vi "TLB Native Dynamic Events ver 0.26.vi"() -> ()   [LabVIEW 2018] (continued)
                      tunnel: string[] ["DISPOSE BUFFERS", "READ STEPPER VALUES", ""] -> [w1790] mode=indexing
                      n604 = Enqueue Element(queue=w1792, element=w1790) -> (queue out=w1791:refnum<queue>)  [unwired: 2 in, 2 out]
                    }
                  }
                }
                n605 = Or(x=w1770, y=w1775) -> (x .or. y?=w1777:bool)
                n606 = Select(t=State_Type_Definitions,_for_0.26g_versions_and_later_2."True Stop" ("Enum"), s=w1775, f=State_Type_Definitions,_for_0.26g_versions_and_later_2."Task 8I: ARM GRAB HEIGHT" ("Enum")) -> (s? t:f=w1772:T16)
                n607 = Select(t=w1772, s=w1777, f=State_Type_Definitions,_for_0.26g_versions_and_later_2."Task 8H: ARM ADJUST" ("Enum")) -> (s? t:f=w1776:T16)
              }
              frame "Exit" {
                n608 = for {
                  shift-right: [w1799] -> w1796
                  shift-left: w1793 -> [w1800]
                  tunnel: string[] ["STOP", "RESET ENCODERS", "RESET YAW", "ARDUINO MODE 0"] -> [w1798] mode=indexing
                  n609 = Enqueue Element(queue=w1800, element=w1798) -> (queue out=w1799:refnum<queue>)  [unwired: 2 in, 2 out]
                }
              }
            }
            n610 = Bundle By Name(cluster=w1759, "yStepper desired"=w1755) -> (w1758:T18)
          }
          frame 35 {
            # ">>> Motor control cluster >>>"
            # ">>> yStepper command>>>"
            # ">> Manual override >>"
            n611 = Dequeue Element(queue=w1811, timeout in ms (-1)=w1810, error in (no error)=w1812) -> (element=w1809:T8)  [unwired: 3 out]
            n612 = Equal?(x=w1808, y=u8 1) -> (x = y?=w1806:bool)
            n613 = case shown="\"Start Task 1\", Default" w1809 {
              tunnel: [w1822 State_Type_Definitions,_for_0.26g_versions_and_later_2."True Stop" ("Enum")] -> w1813
              tunnel: [w1825 w1842] -> w1814
              tunnel: [State_Type_Definitions,_for_0.26g_versions_and_later_2."Idle" ("Enum") State_Type_Definitions,_for_0.26g_versions_and_later_2."Shutdown" ("Enum")] -> w1815
              tunnel: w1806 -> [w1821 _]
              tunnel: w1805 -> [w1820 _]
              tunnel: w1804 -> [w1816 w1839]
              frame "Start Task 1", Default {
                # "Stays in Task 5F until stepper reaches desired \nheight"
                # "T: Go back to idle, F: Continue with task\""
                # ">> Manual override >>"
                n614 = case shown="True" w1821 {
                  tunnel: [w1829 w1835] -> w1825
                  tunnel: w1816 -> [w1827 w1833]
                  frame False {
                    n615 = for {
                      tunnel: string[] ["Z STEPPER GRAB HEIGHT", "READ STEPPER VALUES"] ("element") -> [w1830] mode=indexing
                      shift-right: [w1832] -> w1829
                      shift-left: w1827 -> [w1831]
                      n616 = Enqueue Element(queue=w1831, element=w1830) -> (queue out=w1832:refnum<queue>)  [unwired: 2 in, 2 out]
                    }
                  }
                  frame True {
                    n617 = for {
                      shift-right: [w1837] -> w1835
                      shift-left: w1833 -> [w1838]
                      tunnel: string[] ["SET TIMER 2", "CLOSE CLAW", ""] -> [w1836] mode=indexing
                      n618 = Enqueue Element(queue=w1838, element=w1836) -> (queue out=w1837:refnum<queue>)  [unwired: 2 in, 2 out]
                    }
                  }
                }
                n619 = Or(x=w1821, y=w1820) -> (x .or. y?=w1823:bool)
                n620 = Select(t=State_Type_Definitions,_for_0.26g_versions_and_later_2."True Stop" ("Enum"), s=w1820, f=State_Type_Definitions,_for_0.26g_versions_and_later_2."Task 8J: CLOSE CLAW" ("Enum")) -> (s? t:f=w1817:T16)
                n621 = Select(t=w1817, s=w1823, f=State_Type_Definitions,_for_0.26g_versions_and_later_2."Task 8I: ARM GRAB HEIGHT" ("Enum")) -> (s? t:f=w1822:T16)
              }
              frame "Exit" {
                n622 = for {
                  shift-right: [w1845] -> w1842
                  shift-left: w1839 -> [w1846]
                  tunnel: string[] ["STOP", "RESET ENCODERS", "RESET YAW", "ARDUINO MODE 0"] -> [w1844] mode=indexing
                  n623 = Enqueue Element(queue=w1846, element=w1844) -> (queue out=w1845:refnum<queue>)  [unwired: 2 in, 2 out]
                }
              }
            }
          }
          frame 36 {
            # ">>> yStepper command>>>"
            # ">> Manual override >>"
            n624 = Dequeue Element(queue=w1857, timeout in ms (-1)=w1856, error in (no error)=w1855) -> (element=w1854:T8)  [unwired: 3 out]
            n625 = case shown="\"Start Task 1\", Default" w1854 {
              tunnel: [w1866 State_Type_Definitions,_for_0.26g_versions_and_later_2."True Stop" ("Enum")] -> w1859
              tunnel: [w1869 w1886] -> w1852
              tunnel: [State_Type_Definitions,_for_0.26g_versions_and_later_2."Idle" ("Enum") State_Type_Definitions,_for_0.26g_versions_and_later_2."Shutdown" ("Enum")] -> w1851
              tunnel: w1853 -> [w1860 _]
              tunnel: w1858 -> [w1865 w1883]
              tunnel: w1849 -> [w1864 _]
              frame "Start Task 1", Default {
                # ">> Is time up? >>"
                # "Determines if object is in range to pick up"
                # ">> Manual override >>"
                n626 = case shown="True" w1864 {
                  tunnel: [w1873 w1879] -> w1869
                  tunnel: w1865 -> [w1871 w1877]
                  frame False {
                    n627 = for {
                      tunnel: string[] ["CLOSE CLAW", "START TIMER"] ("element") -> [w1874] mode=indexing
                      shift-right: [w1876] -> w1873
                      shift-left: w1871 -> [w1875]
                      n628 = Enqueue Element(queue=w1875, element=w1874) -> (queue out=w1876:refnum<queue>)  [unwired: 2 in, 2 out]
                    }
                  }
                  frame True {
                    n629 = for {
                      shift-right: [w1881] -> w1879
                      shift-left: w1877 -> [w1882]
                      tunnel: string[] ["READ STEPPER VALUES", "", ""] -> [w1880] mode=indexing
                      n630 = Enqueue Element(queue=w1882, element=w1880) -> (queue out=w1881:refnum<queue>)  [unwired: 2 in, 2 out]
                    }
                  }
                }
                n631 = Or(x=w1864, y=w1860) -> (x .or. y?=w1867:bool)
                n632 = Select(t=State_Type_Definitions,_for_0.26g_versions_and_later_2."True Stop" ("Enum"), s=w1860, f=State_Type_Definitions,_for_0.26g_versions_and_later_2."Task 8K: RAISE MY SWORD" ("Enum")) -> (s? t:f=w1862:T16)
                n633 = Select(t=w1862, s=w1867, f=State_Type_Definitions,_for_0.26g_versions_and_later_2."Task 8J: CLOSE CLAW" ("Enum")) -> (s? t:f=w1866:T16)
              }
              frame "Exit" {
                n634 = for {
                  shift-right: [w1889] -> w1886
                  shift-left: w1883 -> [w1890]
                  tunnel: string[] ["STOP", "RESET ENCODERS", "RESET YAW", "ARDUINO MODE 0"] -> [w1888] mode=indexing
                  n635 = Enqueue Element(queue=w1890, element=w1888) -> (queue out=w1889:refnum<queue>)  [unwired: 2 in, 2 out]
                }
              }
            }
          }
          frame 37 {
            # ">>> yStepper command>>>"
            # ">> Manual override >>"
            n636 = Dequeue Element(queue=w1901, timeout in ms (-1)=w1900, error in (no error)=w1902) -> (element=w1899:T8)  [unwired: 3 out]
            n637 = Equal?(x=w1898, y=u8 60) -> (x = y?=w1896:bool)
            n638 = case shown="\"Start Task 1\", Default" w1899 {
              tunnel: [w1912 State_Type_Definitions,_for_0.26g_versions_and_later_2."True Stop" ("Enum")] -> w1903
              tunnel: [w1915 w1932] -> w1904
              tunnel: [State_Type_Definitions,_for_0.26g_versions_and_later_2."Idle" ("Enum") State_Type_Definitions,_for_0.26g_versions_and_later_2."Shutdown" ("Enum")] -> w1905
              tunnel: w1896 -> [w1911 _]
              tunnel: w1895 -> [w1910 _]
              tunnel: w1894 -> [w1906 w1929]
              frame "Start Task 1", Default {
                # "Stays in Task 5_A until stepper reaches desired \nheight"
                # "T: Go back to idle, F: Continue with task\""
                # ">> Manual override >>"
                n639 = case shown="True" w1911 {
                  tunnel: [w1919 w1925] -> w1915
                  tunnel: w1906 -> [w1917 w1923]
                  frame False {
                    n640 = for {
                      tunnel: string[] ["Z STEPPER CAM HEIGHT", "READ STEPPER VALUES"] ("element") -> [w1920] mode=indexing
                      shift-right: [w1922] -> w1919
                      shift-left: w1917 -> [w1921]
                      n641 = Enqueue Element(queue=w1921, element=w1920) -> (queue out=w1922:refnum<queue>)  [unwired: 2 in, 2 out]
                    }
                  }
                  frame True {
                    n642 = for {
                      shift-right: [w1927] -> w1925
                      shift-left: w1923 -> [w1928]
                      tunnel: string[] ["CAM CLOSE", "DISPOSE CAM BUFFERS", "DISPOSE PROC BUFFERS", "RESET ENCODERS"] -> [w1926] mode=indexing
                      n643 = Enqueue Element(queue=w1928, element=w1926) -> (queue out=w1927:refnum<queue>)  [unwired: 2 in, 2 out]
                    }
                  }
                }
                n644 = Or(x=w1911, y=w1910) -> (x .or. y?=w1913:bool)
                n645 = Select(t=State_Type_Definitions,_for_0.26g_versions_and_later_2."True Stop" ("Enum"), s=w1910, f=State_Type_Definitions,_for_0.26g_versions_and_later_2."True Stop" ("Enum")) -> (s? t:f=w1907:T16)
                n646 = Select(t=w1907, s=w1913, f=State_Type_Definitions,_for_0.26g_versions_and_later_2."Task 8K: RAISE MY SWORD" ("Enum")) -> (s? t:f=w1912:T16)
              }
              frame "Exit" {
                n647 = for {
                  shift-right: [w1935] -> w1932
                  shift-left: w1929 -> [w1936]
                  tunnel: string[] ["STOP", "RESET ENCODERS", "RESET YAW", "ARDUINO MODE 0"] -> [w1934] mode=indexing
                  n648 = Enqueue Element(queue=w1936, element=w1934) -> (queue out=w1935:refnum<queue>)  [unwired: 2 in, 2 out]
                }
              }
            }
          }
          frame 38 {
            # ">>> Motor control cluster >>>"
            # ">> Stepper height reeached >>"
            # ">>> yStepper command>>>"
            # ">> Manual override >>"
            n649 = Dequeue Element(queue=w1948, timeout in ms (-1)=w1943, error in (no error)=w1947) -> (element=w1951:T8)  [unwired: 3 out]
            n650 = Equal?(x=w1945, y=u8 40) -> (x = y?=w1949:bool)
            n651 = case shown="\"Start Task 1\", Default" w1951 {
              tunnel: [w1962 State_Type_Definitions,_for_0.26g_versions_and_later_2."True Stop" ("Enum")] -> w1941
              tunnel: [w1960 w1977] -> w1940
              tunnel: w1944 -> [w1959 _]
              tunnel: w1946 -> [w1953 _]
              tunnel: [State_Type_Definitions,_for_0.26g_versions_and_later_2."Idle" ("Enum") State_Type_Definitions,_for_0.26g_versions_and_later_2."Shutdown" ("Enum")] -> w1942
              tunnel: w1949 -> [w1952 _]
              frame "Start Task 1", Default {
                # ">> WIill proceed to part ii if not manual override >>"
                # ">>If ENABLE or Trigger is set to true>>"
                n652 = Or(x=w1952, y=w1953) -> (x .or. y?=w1954:bool)
                n653 = case shown="True" w1952 {
                  tunnel: [w1965 w1971] -> w1960
                  tunnel: w1959 -> [w1964 w1970]
                  frame False {
                    n654 = for {
                      shift-right: [w1967] -> w1965
                      shift-left: w1964 -> [w1968]
                      tunnel: string[] ["Z STEPPER BOX HEIGHT", "READ STEPPER VALUES"] ("element") -> [w1966] mode=indexing
                      n655 = Enqueue Element(queue=w1968, element=w1966) -> (queue out=w1967:refnum<queue>)  [unwired: 2 in, 2 out]
                    }
                  }
                  frame True {
                    n656 = for {
                      shift-right: [w1973] -> w1971
                      shift-left: w1970 -> [w1974]
                      tunnel: string[] ["ARDUINO - ULTRASONIC", "READ NAVX", "RESET FLAGS", "", "", ""] -> [w1972] mode=indexing
                      n657 = Enqueue Element(queue=w1974, element=w1972) -> (queue out=w1973:refnum<queue>)  [unwired: 2 in, 2 out]
                    }
                  }
                }
                n658 = Select(t=State_Type_Definitions,_for_0.26g_versions_and_later_2."True Stop" ("Enum"), s=w1953, f=State_Type_Definitions,_for_0.26g_versions_and_later_2."Task 9B: Rotate to Angle" ("Enum")) -> (s? t:f=w1956:T16)
                n659 = Select(t=w1956, s=w1954, f=State_Type_Definitions,_for_0.26g_versions_and_later_2."Task 9A: Raise Arm" ("Enum")) -> (s? t:f=w1962:T16)
              }
              frame "Exit" {
                n660 = for {
                  shift-right: [w1980] -> w1977
                  shift-left: _ -> [w1981]
                  tunnel: string[] ["STOP", "RESET ENCODERS", "RESET YAW", ""] -> [w1979] mode=indexing
                  n661 = Enqueue Element(queue=w1981, element=w1979) -> (queue out=w1980:refnum<queue>)  [unwired: 2 in, 2 out]
                }
              }
            }
          }
          frame 39 {
            # ">>> Motor control cluster >>>"
            # ">>> yStepper command>>>"
            n662 = Dequeue Element(queue=w1995, timeout in ms (-1)=w1994, error in (no error)=w1993) -> (element=w1997:T8)  [unwired: 3 out]
            n663 = In Range and Coerce(upper limit=60.0, x=w1987, lower limit=55.0) -> (In Range?=w1984:bool)  [unwired: 1 out]
            n664 = case shown="\"Start Task 1\", Default" w1997 {
              tunnel: w1988 -> [w2000 _]
              tunnel: [w2008 State_Type_Definitions,_for_0.26g_versions_and_later_2."True Stop" ("Enum")] -> w1990
              tunnel: w1996 -> [w2006 w2024]
              tunnel: [w2005 w2023] -> w1989
              tunnel: [State_Type_Definitions,_for_0.26g_versions_and_later_2."Idle" ("Enum") State_Type_Definitions,_for_0.26g_versions_and_later_2."Shutdown" ("Enum")] -> w1991
              tunnel: w1984 -> [w1998 _]
              frame "Start Task 1", Default {
                n665 = Or(x=w1998, y=w2000) -> (x .or. y?=w1999:bool)
                n666 = case shown="True" w1998 {
                  tunnel: w2006 -> [w2011 w2017]
                  tunnel: [w2010 w2015] -> w2005
                  frame False {
                    n667 = for {
                      shift-right: [w2013] -> w2010
                      shift-left: w2011 -> [w2014]
                      tunnel: string[] ["READ NAVX", "R-CW", "READ ULTRASONIC"] ("element") -> [w2012] mode=indexing
                      n668 = Enqueue Element(queue=w2014, element=w2012) -> (queue out=w2013:refnum<queue>)  [unwired: 2 in, 2 out]
                    }
                  }
                  frame True {
                    n669 = for {
                      shift-right: [w2019] -> w2015
                      shift-left: w2017 -> [w2020]
                      tunnel: string[] ["STOP", "RESET ENCODERS", "RESET YAW", "ARDUINO - ULTRASONIC", ""] -> [w2018] mode=indexing
                      n670 = Enqueue Element(queue=w2020, element=w2018) -> (queue out=w2019:refnum<queue>)  [unwired: 2 in, 2 out]
                    }
                  }
                }
                n671 = Select(t=State_Type_Definitions,_for_0.26g_versions_and_later_2."True Stop" ("Enum"), s=w2000, f=State_Type_Definitions,_for_0.26g_versions_and_later_2."Task 9C: Detect Box") -> (s? t:f=w2002:T16)
                n672 = Select(t=w2002, s=w1999, f=State_Type_Definitions,_for_0.26g_versions_and_later_2."Task 9B: Rotate to Angle" ("Enum")) -> (s? t:f=w2008:T16)
              }
              frame "Exit" {
                n673 = for {
                  shift-right: [w2027] -> w2023
                  shift-left: w2024 -> [w2028]
                  tunnel: string[] ["STOP", "RESET ENCODERS", "RESET YAW", ""] -> [w2026] mode=indexing
                  n674 = Enqueue Element(queue=w2028, element=w2026) -> (queue out=w2027:refnum<queue>)  [unwired: 2 in, 2 out]
                }
              }
            }
          }
          frame 40 {
            # ">>> Motor control cluster >>>"
            # ">>Line Detected>>"
            # ">>Action Queue>>"
            # ">>> yStepper command>>>"
            n675 = Dequeue Element(queue=w2040, timeout in ms (-1)=w2039, error in (no error)=w2038) -> (element=w2041:T8)  [unwired: 3 out]
            n676 = case shown="\"Start Task 1\", Default" w2041 {
              tunnel: w2036 -> [w2042 _]
              tunnel: [w2052 State_Type_Definitions,_for_0.26g_versions_and_later_2."True Stop" ("Enum")] -> w2033
              tunnel: w2037 -> [w2050 w2068]
              tunnel: [w2049 w2067] -> w2032
              tunnel: [State_Type_Definitions,_for_0.26g_versions_and_later_2."Idle" ("Enum") State_Type_Definitions,_for_0.26g_versions_and_later_2."Shutdown" ("Enum")] -> w2035
              tunnel: w2030 -> [w2043 _]
              frame "Start Task 1", Default {
                n677 = Or(x=w2042, y=w2043) -> (x .or. y?=w2044:bool)
                n678 = case shown="True" w2043 {
                  tunnel: w2050 -> [w2055 w2061]
                  tunnel: [w2054 w2059] -> w2049
                  frame False {
                    n679 = for {
                      shift-right: [w2057] -> w2054
                      shift-left: w2055 -> [w2058]
                      tunnel: string[] ["READ IR", "READ LINE SENSOR", "FORWARD - IR ASSIST"] ("element") -> [w2056] mode=indexing
                      n680 = Enqueue Element(queue=w2058, element=w2056) -> (queue out=w2057:refnum<queue>)  [unwired: 2 in, 2 out]
                    }
                  }
                  frame True {
                    n681 = for {
                      shift-right: [w2063] -> w2059
                      shift-left: w2061 -> [w2064]
                      tunnel: string[] ["STOP", "RESET ENCODERS", "RESET YAW", ""] -> [w2062] mode=indexing
                      n682 = Enqueue Element(queue=w2064, element=w2062) -> (queue out=w2063:refnum<queue>)  [unwired: 2 in, 2 out]
                    }
                  }
                }
                n683 = Select(t=State_Type_Definitions,_for_0.26g_versions_and_later_2."True Stop" ("Enum"), s=w2042, f=State_Type_Definitions,_for_0.26g_versions_and_later_2."Task 9D: MOVE FORWARD") -> (s? t:f=w2046:T16)
                n684 = Select(t=w2046, s=w2044, f=State_Type_Definitions,_for_0.26g_versions_and_later_2."Task 9C: Detect Box" ("Enum")) -> (s? t:f=w2052:T16)
              }
              frame "Exit" {
                n685 = for {
                  shift-right: [w2071] -> w2067
                  shift-left: w2068 -> [w2072]
                  tunnel: string[] ["STOP", "RESET ENCODERS", "RESET YAW", ""] -> [w2070] mode=indexing
                  n686 = Enqueue Element(queue=w2072, element=w2070) -> (queue out=w2071:refnum<queue>)  [unwired: 2 in, 2 out]
                }
              }
            }
          }
          frame 41 {
            # ">> Item Selection Bias >>"
            # ">> Wall detected >>"
            # ">> Manual override >>"
            # ">>Table Detected>>"
            # ">>> Motor control cluster >>>"
            # ">>Table or wall detectected>>"
            # ">>Action Queue>>"
            # ">>> yStepper command>>>"
            n687 = Dequeue Element(queue=w2090, timeout in ms (-1)=w2089, error in (no error)=w2088) -> (element=w2091:T8)  [unwired: 3 out]
            n688 = Less Or Equal?(x=w2079, y=15.0) -> (x <= y?=w2073:bool)
            n689 = Less?(x=w2076, y=182.0) -> (x < y?=w2074:bool)
            n690 = Or(x=w2073, y=w2074) -> (x .or. y?=w2077:bool)
            n691 = case shown="\"Start Task 1\", Default" w2091 {
              tunnel: w2086 -> [w2092 _]
              tunnel: [w2102 State_Type_Definitions,_for_0.26g_versions_and_later_2."True Stop" ("Enum")] -> w2083
              tunnel: w2087 -> [w2100 w2118]
              tunnel: [w2099 w2117] -> w2082
              tunnel: [State_Type_Definitions,_for_0.26g_versions_and_later_2."Idle" ("Enum") State_Type_Definitions,_for_0.26g_versions_and_later_2."Shutdown" ("Enum")] -> w2085
              tunnel: w2077 -> [w2093 _]
              frame "Start Task 1", Default {
                n692 = Or(x=w2092, y=w2093) -> (x .or. y?=w2094:bool)
                n693 = case shown="False" w2093 {
                  tunnel: w2100 -> [w2105 w2111]
                  tunnel: [w2104 w2109] -> w2099
                  frame False {
                    n694 = for {
                      shift-right: [w2107] -> w2104
                      shift-left: w2105 -> [w2108]
                      tunnel: string[] ["READ IR", "FORWARD - IR ASSIST", "READ ULTRASONIC"] ("element") -> [w2106] mode=indexing
                      n695 = Enqueue Element(queue=w2108, element=w2106) -> (queue out=w2107:refnum<queue>)  [unwired: 2 in, 2 out]
                    }
                  }
                  frame True {
                    n696 = for {
                      shift-right: [w2113] -> w2109
                      shift-left: w2111 -> [w2114]
                      tunnel: string[] ["STOP", "RESET ENCODERS", "RESET YAW", ""] -> [w2112] mode=indexing
                      n697 = Enqueue Element(queue=w2114, element=w2112) -> (queue out=w2113:refnum<queue>)  [unwired: 2 in, 2 out]
                    }
                  }
                }
                n698 = Select(t=State_Type_Definitions,_for_0.26g_versions_and_later_2."True Stop" ("Enum"), s=w2092, f=State_Type_Definitions,_for_0.26g_versions_and_later_2."Task 9E: MOVE LEFT") -> (s? t:f=w2096:T16)
                n699 = Select(t=w2096, s=w2094, f=State_Type_Definitions,_for_0.26g_versions_and_later_2."Task 9D: MOVE FORWARD" ("Enum")) -> (s? t:f=w2102:T16)
              }
              frame "Exit" {
                n700 = for {
                  shift-right: [w2121] -> w2117
                  shift-left: w2118 -> [w2122]
                  tunnel: string[] ["STOP", "RESET ENCODERS", "RESET YAW", ""] -> [w2120] mode=indexing
                  n701 = Enqueue Element(queue=w2122, element=w2120) -> (queue out=w2121:refnum<queue>)  [unwired: 2 in, 2 out]
                }
              }
            }
          }
          frame 42 {
            # ">> Item Selection Bias >>"
            # ">> Line detected? >>"
            # ">> Manual override >>"
            # ">>> Motor control cluster >>>"
            # ">>Action Queue>>"
            # ">>> yStepper command>>>"
            n702 = Dequeue Element(queue=w2134, timeout in ms (-1)=w2133, error in (no error)=w2132) -> (element=w2135:T8)  [unwired: 3 out]
            n703 = case shown="\"Start Task 1\", Default" w2135 {
              tunnel: w2130 -> [w2136 _]
              tunnel: [w2146 State_Type_Definitions,_for_0.26g_versions_and_later_2."True Stop" ("Enum")] -> w2127
              tunnel: w2131 -> [w2144 w2162]
              tunnel: [w2143 w2161] -> w2126
              tunnel: [State_Type_Definitions,_for_0.26g_versions_and_later_2."Idle" ("Enum") State_Type_Definitions,_for_0.26g_versions_and_later_2."Shutdown" ("Enum")] -> w2129
              tunnel: w2123 -> [w2137 _]
              frame "Start Task 1", Default {
                n704 = Or(x=w2136, y=w2137) -> (x .or. y?=w2138:bool)
                n705 = case shown="False" w2137 {
                  tunnel: w2144 -> [w2149 w2155]
                  tunnel: [w2148 w2153] -> w2143
                  frame False {
                    n706 = for {
                      shift-right: [w2151] -> w2148
                      shift-left: w2149 -> [w2152]
                      tunnel: string[] ["LEFT", "READ NAVX", "READ LINE SENSOR", ""] ("element") -> [w2150] mode=indexing
                      n707 = Enqueue Element(queue=w2152, element=w2150) -> (queue out=w2151:refnum<queue>)  [unwired: 2 in, 2 out]
                    }
                  }
                  frame True {
                    n708 = for {
                      shift-right: [w2157] -> w2153
                      shift-left: w2155 -> [w2158]
                      tunnel: string[] ["STOP", "RESET ENCODERS", "RESET YAW", "RESET FLAGS", "OPEN LIFE CAM", "SET TIMER 2"] -> [w2156] mode=indexing
                      n709 = Enqueue Element(queue=w2158, element=w2156) -> (queue out=w2157:refnum<queue>)  [unwired: 2 in, 2 out]
                    }
                  }
                }
                n710 = Select(t=State_Type_Definitions,_for_0.26g_versions_and_later_2."True Stop" ("Enum"), s=w2136, f=State_Type_Definitions,_for_0.26g_versions_and_later_2."True Stop") -> (s? t:f=w2140:T16)
                n711 = Select(t=w2140, s=w2138, f=State_Type_Definitions,_for_0.26g_versions_and_later_2."Task 9E: MOVE LEFT" ("Enum")) -> (s? t:f=w2146:T16)
              }
              frame "Exit" {
                n712 = for {
                  shift-right: [w2165] -> w2161
                  shift-left: w2162 -> [w2166]
                  tunnel: string[] ["STOP", "RESET ENCODERS", "RESET YAW", ""] -> [w2164] mode=indexing
                  n713 = Enqueue Element(queue=w2166, element=w2164) -> (queue out=w2165:refnum<queue>)  [unwired: 2 in, 2 out]
                }
              }
            }
          }
          frame 43 {
            # ">>> Motor control cluster >>>"
            # ">>Time up? >>"
            # ">>> yStepper command>>>"
            # ">> Manual override >>"
            n714 = Dequeue Element(queue=w2178, timeout in ms (-1)=w2174, error in (no error)=w2177) -> (element=w2179:T8)  [unwired: 3 out]
            n715 = case shown="\"Start Task 1\", Default" w2179 {
              tunnel: [w2190 State_Type_Definitions,_for_0.26g_versions_and_later_2."True Stop" ("Enum")] -> w2172
              tunnel: [w2188 w2206] -> w2171
              tunnel: w2175 -> [w2187 w2203]
              tunnel: w2176 -> [w2181 _]
              tunnel: [State_Type_Definitions,_for_0.26g_versions_and_later_2."Idle" ("Enum") State_Type_Definitions,_for_0.26g_versions_and_later_2."Shutdown" ("Enum")] -> w2173
              tunnel: w2167 -> [w2180 _]
              frame "Start Task 1", Default {
                # ">> WIill proceed to part ii if not manual override >>"
                # ">>If ENABLE or Trigger is set to true>>"
                n716 = Or(x=w2180, y=w2181) -> (x .or. y?=w2182:bool)
                n717 = case shown="True" w2180 {
                  tunnel: [w2193 w2199] -> w2188
                  tunnel: w2187 -> [w2192 w2198]
                  frame False {
                    n718 = for {
                      shift-right: [w2195] -> w2193
                      shift-left: w2192 -> [w2196]
                      tunnel: string[] ["CAM ACQ", "START TIMER"] ("element") -> [w2194] mode=indexing
                      n719 = Enqueue Element(queue=w2196, element=w2194) -> (queue out=w2195:refnum<queue>)  [unwired: 2 in, 2 out]
                    }
                  }
                  frame True {
                    n720 = for {
                      shift-right: [w2201] -> w2199
                      shift-left: w2198 -> [w2202]
                      tunnel: string[] ["CLOSE CAM", "SET TIMER 5", "", "", "", ""] -> [w2200] mode=indexing
                      n721 = Enqueue Element(queue=w2202, element=w2200) -> (queue out=w2201:refnum<queue>)  [unwired: 2 in, 2 out]
                    }
                  }
                }
                n722 = Select(t=State_Type_Definitions,_for_0.26g_versions_and_later_2."True Stop" ("Enum"), s=w2181, f=State_Type_Definitions."Task 9G: PROCESS COLOUR" ("Enum")) -> (s? t:f=w2184:u16)
                n723 = Select(t=w2184, s=w2182, f=State_Type_Definitions."Task 9F: SCAN IMAGE" ("Enum")) -> (s? t:f=w2190:u16)
              }
              frame "Exit" {
                n724 = for {
                  shift-right: [w2209] -> w2206
                  shift-left: w2203 -> [w2210]
                  tunnel: string[] ["STOP", "RESET ENCODERS", "RESET YAW", ""] -> [w2208] mode=indexing
                  n725 = Enqueue Element(queue=w2210, element=w2208) -> (queue out=w2209:refnum<queue>)  [unwired: 2 in, 2 out]
                }
              }
            }
          }
          frame 44 {
            # ">>> Motor control cluster >>>"
            # ">>> yStepper command>>>"
            # ">>Object detected>>"
            n726 = Less Or Equal?(x=w2214, y=30.0) -> (x <= y?=w2212:bool)
            "Table obstruct" <- w2212
            n727 = Dequeue Element(queue=w2220, timeout in ms (-1)=w2219, error in (no error)=w2218) -> (element=w2225:T8)  [unwired: 3 out]
            n728 = case shown="\"Start Task 1\", Default" w2225 {
              tunnel: w2212 -> [w2228 _]
              tunnel: [w2235 State_Type_Definitions,_for_0.26g_versions_and_later_2."True Stop" ("Enum")] -> w2224
              tunnel: w2217 -> [w2227 _]
              tunnel: w2221 -> [w2234 w2251]
              tunnel: [w2233 w2252] -> w2223
              tunnel: [State_Type_Definitions,_for_0.26g_versions_and_later_2."Idle" ("Enum") State_Type_Definitions,_for_0.26g_versions_and_later_2."Shutdown" ("Enum")] -> w2222
              frame "Start Task 1", Default {
                n729 = case shown="True" w2228 {
                  tunnel: w2234 -> [w2238 w2245]
                  tunnel: [w2239 w2244] -> w2233
                  frame False {
                    n730 = for {
                      tunnel: string[] ["START TIMER", "COLOUR PROCESSING", ""] ("element") -> [w2240] mode=indexing
                      shift-right: [w2242] -> w2239
                      shift-left: w2238 -> [w2241]
                      n731 = Enqueue Element(queue=w2241, element=w2240) -> (queue out=w2242:refnum<queue>)  [unwired: 2 in, 2 out]
                    }
                  }
                  frame True {
                    n732 = for {
                      shift-right: [w2247] -> w2244
                      shift-left: w2245 -> [w2248]
                      tunnel: string[] ["DISPOSE BUFFERS", "CLOSE CAM", "RESET ENCODERS", "RESET YAW", "RESET FLAGS"] -> [w2246] mode=indexing
                      n733 = Enqueue Element(queue=w2248, element=w2246) -> (queue out=w2247:refnum<queue>)  [unwired: 2 in, 2 out]
                    }
                  }
                }
                n734 = Or(x=w2228, y=w2227) -> (x .or. y?=w2226:bool)
                n735 = Select(t=State_Type_Definitions,_for_0.26g_versions_and_later_2."True Stop" ("Enum"), s=w2227, f=State_Type_Definitions."Task 9H: MOVE RIGHT" ("Enum")) -> (s? t:f=w2229:u16)
                n736 = Select(t=w2229, s=w2226, f=State_Type_Definitions."Task 9G: PROCESS COLOUR" ("Enum")) -> (s? t:f=w2235:u16)
              }
              frame "Exit" {
                n737 = for {
                  shift-right: [w2255] -> w2252
                  shift-left: w2251 -> [w2256]
                  tunnel: string[] ["STOP", "RESET ENCODERS", "RESET YAW", "ARDUINO MODE 0"] -> [w2254] mode=indexing
                  n738 = Enqueue Element(queue=w2256, element=w2254) -> (queue out=w2255:refnum<queue>)  [unwired: 2 in, 2 out]
                }
              }
            }
          }
          frame 45 {
            # ">> Item Selection Bias >>"
            # ">>> Motor control cluster >>>"
            # ">>> yStepper command>>>"
            n739 = Dequeue Element(queue=w2266, timeout in ms (-1)=w2267, error in (no error)=w2268) -> (element=w2270:T8)  [unwired: 3 out]
            n740 = Greater?(x=w2258, y=50.0) -> (0:w2259:bool)
            n741 = And(x=w2260, y=w2259) -> (x .and. y?=w2261:bool)
            n742 = case shown="\"Start Task 1\", Default" w2270 {
              tunnel: w2261 -> [w2276 _]
              tunnel: [w2283 State_Type_Definitions,_for_0.26g_versions_and_later_2."True Stop" ("Enum")] -> w2263
              tunnel: w2269 -> [w2275 _]
              tunnel: w2265 -> [w2282 w2299]
              tunnel: [w2281 w2300] -> w2264
              tunnel: [State_Type_Definitions,_for_0.26g_versions_and_later_2."Idle" ("Enum") State_Type_Definitions,_for_0.26g_versions_and_later_2."Shutdown" ("Enum")] -> w2262
              frame "Start Task 1", Default {
                n743 = case shown="False" w2276 {
                  tunnel: w2282 -> [w2286 w2293]
                  tunnel: [w2287 w2292] -> w2281
                  frame False {
                    n744 = for {
                      tunnel: string[] ["READ LINE SENSOR", "READ NAVX", "RIGHT", "READ ENCODERS"] ("element") -> [w2288] mode=indexing
                      shift-right: [w2290] -> w2287
                      shift-left: w2286 -> [w2289]
                      n745 = Enqueue Element(queue=w2289, element=w2288) -> (queue out=w2290:refnum<queue>)  [unwired: 2 in, 2 out]
                    }
                  }
                  frame True {
                    n746 = for {
                      shift-right: [w2295] -> w2292
                      shift-left: w2293 -> [w2296]
                      tunnel: string[] ["STOP", "RESET ENCODERS", "RESET YAW", "OPEN LIFE CAM", "SET TIMER 2", "RESET FLAGS"] -> [w2294] mode=indexing
                      n747 = Enqueue Element(queue=w2296, element=w2294) -> (queue out=w2295:refnum<queue>)  [unwired: 2 in, 2 out]
                    }
                  }
                }
                n748 = Or(x=w2276, y=w2275) -> (x .or. y?=w2274:bool)
                n749 = Select(t=State_Type_Definitions,_for_0.26g_versions_and_later_2."True Stop" ("Enum"), s=w2275, f=State_Type_Definitions."Task 9I: SCAN IMAGE" ("Enum")) -> (s? t:f=w2277:u16)
                n750 = Select(t=w2277, s=w2274, f=State_Type_Definitions."Task 9H: MOVE RIGHT" ("Enum")) -> (s? t:f=w2283:u16)
              }
              frame "Exit" {
                n751 = for {
                  shift-right: [w2303] -> w2300
                  shift-left: w2299 -> [w2304]
                  tunnel: string[] ["STOP", "RESET ENCODERS", "RESET YAW", "ARDUINO MODE 0"] -> [w2302] mode=indexing
                  n752 = Enqueue Element(queue=w2304, element=w2302) -> (queue out=w2303:refnum<queue>)  [unwired: 2 in, 2 out]
                }
              }
            }
          }
          frame 46 {
            # ">> Item Selection Bias >>"
            n753 = Dequeue Element(queue=w2306, timeout in ms (-1)=w2307, error in (no error)=w2308) -> (element=w2314:T8)  [unwired: 3 out]
            n754 = case shown="\"Start Task 1\", Default" w2314 {
              tunnel: w2305 -> [w2320 _]
              tunnel: [w2327 State_Type_Definitions,_for_0.26g_versions_and_later_2."True Stop" ("Enum")] -> w2311
              tunnel: w2309 -> [w2319 _]
              tunnel: w2313 -> [w2326 w2343]
              tunnel: [w2325 w2344] -> w2312
              tunnel: [State_Type_Definitions,_for_0.26g_versions_and_later_2."Idle" ("Enum") State_Type_Definitions,_for_0.26g_versions_and_later_2."Shutdown" ("Enum")] -> w2310
              frame "Start Task 1", Default {
                n755 = case shown="True" w2320 {
                  tunnel: w2326 -> [w2330 w2337]
                  tunnel: [w2331 w2336] -> w2325
                  frame False {
                    n756 = for {
                      tunnel: string[] ["START TIMER", "CAM ACQ", ""] ("element") -> [w2332] mode=indexing
                      shift-right: [w2334] -> w2331
                      shift-left: w2330 -> [w2333]
                      n757 = Enqueue Element(queue=w2333, element=w2332) -> (queue out=w2334:refnum<queue>)  [unwired: 2 in, 2 out]
                    }
                  }
                  frame True {
                    n758 = for {
                      shift-right: [w2339] -> w2336
                      shift-left: w2337 -> [w2340]
                      tunnel: string[] ["CLOSE CAM", "SET TIMER 5", "", "", "", ""] -> [w2338] mode=indexing
                      n759 = Enqueue Element(queue=w2340, element=w2338) -> (queue out=w2339:refnum<queue>)  [unwired: 2 in, 2 out]
                    }
                  }
                }
                n760 = Or(x=w2320, y=w2319) -> (x .or. y?=w2318:bool)
                n761 = Select(t=State_Type_Definitions,_for_0.26g_versions_and_later_2."True Stop" ("Enum"), s=w2319, f=State_Type_Definitions."Task 9J: PROCESS COLOUR" ("Enum")) -> (s? t:f=w2321:u16)
                n762 = Select(t=w2321, s=w2318, f=State_Type_Definitions."Task 9I: SCAN IMAGE" ("Enum")) -> (s? t:f=w2327:u16)
              }
              frame "Exit" {
                n763 = for {
                  shift-right: [w2347] -> w2344
                  shift-left: w2343 -> [w2348]
                  tunnel: string[] ["STOP", "RESET ENCODERS", "RESET YAW", "ARDUINO MODE 0"] -> [w2346] mode=indexing
                  n764 = Enqueue Element(queue=w2348, element=w2346) -> (queue out=w2347:refnum<queue>)  [unwired: 2 in, 2 out]
                }
              }
            }
          }
          frame 47 {
            # ">> Item Selection Bias >>"
            n765 = Dequeue Element(queue=w2354, timeout in ms (-1)=w2355, error in (no error)=w2356) -> (element=w2358:T8)  [unwired: 3 out]
            n766 = case shown="\"Start Task 1\", Default" w2358 {
              tunnel: w2349 -> [w2364 _]
              tunnel: [w2371 State_Type_Definitions,_for_0.26g_versions_and_later_2."True Stop" ("Enum")] -> w2352
              tunnel: w2357 -> [w2363 _]
              tunnel: w2353 -> [w2370 w2387]
              tunnel: [w2369 w2388] -> w2351
              tunnel: [State_Type_Definitions,_for_0.26g_versions_and_later_2."Idle" ("Enum") State_Type_Definitions,_for_0.26g_versions_and_later_2."Shutdown" ("Enum")] -> w2350
              frame "Start Task 1", Default {
                n767 = case shown="True" w2364 {
                  tunnel: w2370 -> [w2374 w2381]
                  tunnel: [w2375 w2380] -> w2369
                  frame False {
                    n768 = for {
                      tunnel: string[] ["START TIMER", "COLOUR PROCESSING", ""] ("element") -> [w2376] mode=indexing
                      shift-right: [w2378] -> w2375
                      shift-left: w2374 -> [w2377]
                      n769 = Enqueue Element(queue=w2377, element=w2376) -> (queue out=w2378:refnum<queue>)  [unwired: 2 in, 2 out]
                    }
                  }
                  frame True {
                    n770 = for {
                      shift-right: [w2383] -> w2380
                      shift-left: w2381 -> [w2384]
                      tunnel: string[] ["CLOSE CAM", "DISPOSE BUFFERS", "RESET ENCODERS", "RESET YAW", "RESET FLAGS", ""] -> [w2382] mode=indexing
                      n771 = Enqueue Element(queue=w2384, element=w2382) -> (queue out=w2383:refnum<queue>)  [unwired: 2 in, 2 out]
                    }
                  }
                }
                n772 = Or(x=w2364, y=w2363) -> (x .or. y?=w2362:bool)
                n773 = Select(t=State_Type_Definitions,_for_0.26g_versions_and_later_2."True Stop" ("Enum"), s=w2363, f=State_Type_Definitions."Task 9K: ROTATE 90 CW" ("Enum")) -> (s? t:f=w2365:u16)
                n774 = Select(t=w2365, s=w2362, f=State_Type_Definitions."Task 9J: PROCESS COLOUR" ("Enum")) -> (s? t:f=w2371:u16)
              }
              frame "Exit" {
                n775 = for {
                  shift-right: [w2391] -> w2388
                  shift-left: w2387 -> [w2392]
                  tunnel: string[] ["STOP", "RESET ENCODERS", "RESET YAW", "ARDUINO MODE 0"] -> [w2390] mode=indexing
                  n776 = Enqueue Element(queue=w2392, element=w2390) -> (queue out=w2391:refnum<queue>)  [unwired: 2 in, 2 out]
                }
              }
            }
          }
          frame 48 {
            # ">>> Motor control cluster >>>"
            # ">>> yStepper command>>>"
            # ">> Item Selection Bias >>"
            n777 = Less?(x=w2396, y=-38.0) -> (x < y?=w2394:bool)
            n778 = Dequeue Element(queue=w2402, timeout in ms (-1)=w2401, error in (no error)=w2400) -> (element=w2404:T8)  [unwired: 3 out]
            n779 = case shown="\"Start Task 1\", Default" w2404 {
              tunnel: w2394 -> [w2410 _]
              tunnel: [w2417 State_Type_Definitions,_for_0.26g_versions_and_later_2."True Stop" ("Enum")] -> w2398
              tunnel: w2399 -> [w2409 _]
              tunnel: w2403 -> [w2416 w2433]
              tunnel: [w2415 w2434] -> w2393
              tunnel: [State_Type_Definitions,_for_0.26g_versions_and_later_2."Idle" ("Enum") State_Type_Definitions,_for_0.26g_versions_and_later_2."Shutdown" ("Enum")] -> w2397
              frame "Start Task 1", Default {
                n780 = case shown="True" w2410 {
                  tunnel: w2416 -> [w2420 w2427]
                  tunnel: [w2421 w2426] -> w2415
                  frame False {
                    n781 = for {
                      tunnel: string[] ["READ ENCODERS", "R-CW"] ("element") -> [w2422] mode=indexing
                      shift-right: [w2424] -> w2421
                      shift-left: w2420 -> [w2423]
                      n782 = Enqueue Element(queue=w2423, element=w2422) -> (queue out=w2424:refnum<queue>)  [unwired: 2 in, 2 out]
                    }
                  }
                  frame True {
                    n783 = for {
                      shift-right: [w2429] -> w2426
                      shift-left: w2427 -> [w2430]
                      tunnel: string[] ["STOP", "RESET ENCODERS", "RESET FLAGS", "RESET YAW", "READ IR", "ARDUINO - ULTRASONIC"] -> [w2428] mode=indexing
                      n784 = Enqueue Element(queue=w2430, element=w2428) -> (queue out=w2429:refnum<queue>)  [unwired: 2 in, 2 out]
                    }
                  }
                }
                n785 = Or(x=w2410, y=w2409) -> (x .or. y?=w2408:bool)
                n786 = Select(t=State_Type_Definitions,_for_0.26g_versions_and_later_2."True Stop" ("Enum"), s=w2409, f=State_Type_Definitions."Task 9L: MOVE FORWARD" ("Enum")) -> (s? t:f=w2411:u16)
                n787 = Select(t=w2411, s=w2408, f=State_Type_Definitions."Task 9K: ROTATE 90 CW" ("Enum")) -> (s? t:f=w2417:u16)
              }
              frame "Exit" {
                n788 = for {
                  shift-right: [w2437] -> w2434
                  shift-left: w2433 -> [w2438]
                  tunnel: string[] ["STOP", "RESET ENCODERS", "RESET YAW", "ARDUINO MODE 0"] -> [w2436] mode=indexing
                  n789 = Enqueue Element(queue=w2438, element=w2436) -> (queue out=w2437:refnum<queue>)  [unwired: 2 in, 2 out]
                }
              }
            }
          }
          frame 49 {
            w2451 = u8 50 ("y")
            # ">>> Motor control cluster >>>"
            # ">>> yStepper command>>>"
            # ">> Item Selection Bias >>"
            n790 = Less?(x=w2453, y=w2451) -> (x < y?=w2446:bool)
            n791 = Dequeue Element(queue=w2457, timeout in ms (-1)=w2456, error in (no error)=w2455) -> (element=w2461:T8)  [unwired: 3 out]
            n792 = Less?(x=w2452, y=w2451) -> (x < y?=w2447:bool)
            n793 = And(x=w2447, y=w2446) -> (x .and. y?=w2439:bool)
            n794 = Less Or Equal?(x=w2450, y=15.0) -> (x <= y?=w2445:bool)
            n795 = Greater?(x=w2444, y=100.0) -> (0:w2443:bool)
            n796 = Or(x=w2445, y=w2439) -> (x .or. y?=w2441:bool)
            n797 = And(x=w2443, y=w2441) -> (x .and. y?=w2442:bool)
            n798 = case shown="\"Start Task 1\", Default" w2461 {
              tunnel: w2442 -> [w2467 _]
              tunnel: [w2474 State_Type_Definitions,_for_0.26g_versions_and_later_2."True Stop" ("Enum")] -> w2459
              tunnel: w2454 -> [w2466 _]
              tunnel: w2458 -> [w2473 w2490]
              tunnel: [w2472 w2491] -> w2448
              tunnel: [State_Type_Definitions,_for_0.26g_versions_and_later_2."Idle" ("Enum") State_Type_Definitions,_for_0.26g_versions_and_later_2."Shutdown" ("Enum")] -> w2460
              frame "Start Task 1", Default {
                n799 = case shown="True" w2467 {
                  tunnel: w2473 -> [w2477 w2484]
                  tunnel: [w2478 w2483] -> w2472
                  frame False {
                    n800 = for {
                      tunnel: string[] ["READ IR", "FORWARD", "READ NAVX", "READ ENCODERS"] ("element") -> [w2479] mode=indexing
                      shift-right: [w2481] -> w2478
                      shift-left: w2477 -> [w2480]
                      n801 = Enqueue Element(queue=w2480, element=w2479) -> (queue out=w2481:refnum<queue>)  [unwired: 2 in, 2 out]
                    }
                  }
                  frame True {
                    n802 = for {
                      shift-right: [w2486] -> w2483
                      shift-left: w2484 -> [w2487]
                      tunnel: string[] ["STOP", "RESET ENCODERS", "RESET FLAGS", "RESET YAW", "", ""] -> [w2485] mode=indexing
                      n803 = Enqueue Element(queue=w2487, element=w2485) -> (queue out=w2486:refnum<queue>)  [unwired: 2 in, 2 out]
                    }
                  }
                }
                n804 = Or(x=w2467, y=w2466) -> (x .or. y?=w2465:bool)
                n805 = Select(t=State_Type_Definitions,_for_0.26g_versions_and_later_2."True Stop" ("Enum"), s=w2466, f=State_Type_Definitions,_for_0.26g_versions_and_later_2."True Stop" ("Enum")) -> (s? t:f=w2468:T16)
                n806 = Select(t=w2468, s=w2465, f=State_Type_Definitions."Task 9L: MOVE FORWARD" ("Enum")) -> (s? t:f=w2474:u16)
              }
              frame "Exit" {
                n807 = for {
                  shift-right: [w2494] -> w2491
                  shift-left: w2490 -> [w2495]
                  tunnel: string[] ["STOP", "RESET ENCODERS", "RESET YAW", "ARDUINO MODE 0"] -> [w2493] mode=indexing
                  n808 = Enqueue Element(queue=w2495, element=w2493) -> (queue out=w2494:refnum<queue>)  [unwired: 2 in, 2 out]
                }
              }
            }
          }
          frame 50 {
            # ">> Item Selection Bias >>"
            n809 = Dequeue Element(queue=w2500, timeout in ms (-1)=w2499, error in (no error)=w2498) -> (element=w2505:T8)  [unwired: 3 out]
            n810 = case shown="\"Start Task 1\", Default" w2505 {
              tunnel: w2496 -> [w2511 _]
              tunnel: [w2518 State_Type_Definitions,_for_0.26g_versions_and_later_2."True Stop" ("Enum")] -> w2503
              tunnel: w2497 -> [w2510 _]
              tunnel: w2501 -> [w2517 w2534]
              tunnel: [w2516 w2535] -> w2502
              tunnel: [State_Type_Definitions,_for_0.26g_versions_and_later_2."Idle" ("Enum") State_Type_Definitions,_for_0.26g_versions_and_later_2."Shutdown" ("Enum")] -> w2504
              frame "Start Task 1", Default {
                n811 = case shown="False" w2511 {
                  tunnel: w2517 -> [w2521 w2528]
                  tunnel: [w2522 w2527] -> w2516
                  frame False {
                    n812 = for {
                      tunnel: string[] ["READ LINE SENSOR", "READ NAVX", "RIGHT", "READ ENCODERS"] ("element") -> [w2523] mode=indexing
                      shift-right: [w2525] -> w2522